vi "HFRR ADV v041.vi"() -> ()   [LabVIEW 2025] (continued)
            n2218 = Delete From Array(array=w2421, index=0) -> (array with subset deleted=w2408:dbl[])  [unwired: 1 in, 1 out]
            n2219 = Delete From Array(array=w2461, index=0) -> (array with subset deleted=w2432:dbl[])  [unwired: 1 in, 1 out]
            n2220 = Delete From Array(array=w2539, index=0) -> (array with subset deleted=w2494:dbl[])  [unwired: 1 in, 1 out]
            n2221 = Delete From Array(array=w2505, index=0) -> (array with subset deleted=w2490:dbl[])  [unwired: 1 in, 1 out]
            "array w/ subset deleted" <- w2490
            n2222 = Delete From Array(array=w2536, index=0) -> (array with subset deleted=w2537:dbl[])  [unwired: 1 in, 1 out]
            n2223 = call-poly <vilib>:"Mean.vi"("X"=w2432) -> ("mean"=→"КОФ2 2":dbl)  [unwired: 1 out]
            n2224 = call-poly <vilib>:"Mean.vi"("X"=w2494) -> ("mean"=→"КОФ1":dbl)  [unwired: 1 out]
            n2225 = Bundle "Bundle"(w2409, w2408) -> (w2414:cluster{dbl[], dbl[]})  [unwired: 1 in]
            n2226 = Bundle "Bundle"(w2409, w2537) -> (w2401:cluster{dbl[], dbl[]})  [unwired: 1 in]
            n2227 = Delete From Array(array=w2416, index=0) -> (array with subset deleted=w2404:dbl[])  [unwired: 1 in, 1 out]
            n2228 = Delete From Array(array=w2417, index=0) -> (array with subset deleted=w2406:dbl[])  [unwired: 1 in, 1 out]
            n2229 = Delete From Array(array=w2527, index=0) -> (array with subset deleted=w2528:dbl[])  [unwired: 1 in, 1 out]
            n2230 = Delete From Array(array=w2415, index=0) -> (array with subset deleted=w2402:dbl[])  [unwired: 1 in, 1 out]
            n2231 = Delete From Array(array=w2509, index=0) -> (array with subset deleted=w2510:dbl[])  [unwired: 1 in, 1 out]
            n2232 = Delete From Array(array=w2534, index=0) -> (array with subset deleted=w2440:dbl[])  [unwired: 1 in, 1 out]
            n2233 = Delete From Array(array=w2480, index=0) -> (array with subset deleted=w2436:dbl[])  [unwired: 1 in, 1 out]
            n2234 = Delete From Array(array=w2516, index=0) -> (array with subset deleted=w2438:dbl[])  [unwired: 1 in, 1 out]
            n2235 = Delete From Array(array=w2476, index=0) -> (array with subset deleted=w2434:dbl[])  [unwired: 1 in, 1 out]
            n2236 = Delete From Array(array=w2525, index=0) -> (array with subset deleted=w2439:dbl[])  [unwired: 1 in, 1 out]
            n2237 = Delete From Array(array=w2478, index=0) -> (array with subset deleted=w2435:dbl[])  [unwired: 1 in, 1 out]
            n2238 = Delete From Array(array=w2459, index=0) -> (array with subset deleted=w2431:dbl[])  [unwired: 1 in, 1 out]
            n2239 = Delete From Array(array=w2503, index=0) -> (array with subset deleted=w2489:dbl[])  [unwired: 1 in, 1 out]
            n2240 = Delete From Array(array=w2530, index=0) -> (array with subset deleted=w2491:dbl[])  [unwired: 1 in, 1 out]
            n2241 = Delete From Array(array=w2507, index=0) -> (array with subset deleted=w2437:dbl[])  [unwired: 1 in, 1 out]
            n2242 = Delete From Array(array=w2474, index=0) -> (array with subset deleted=w2433:dbl[])  [unwired: 1 in, 1 out]
            n2243 = Delete From Array(array=w2455, index=0) -> (array with subset deleted=w2429:dbl[])  [unwired: 1 in, 1 out]
            n2244 = Delete From Array(array=w2499, index=0) -> (array with subset deleted=w2487:dbl[])  [unwired: 1 in, 1 out]
            n2245 = Delete From Array(array=w2512, index=0) -> (array with subset deleted=w2492:dbl[])  [unwired: 1 in, 1 out]
            n2246 = Delete From Array(array=w2522, index=0) -> (array with subset deleted=w2405:dbl[])  [unwired: 1 in, 1 out]
            n2247 = Delete From Array(array=w2532, index=0) -> (array with subset deleted=w2407:dbl[])  [unwired: 1 in, 1 out]
            n2248 = Delete From Array(array=w2514, index=0) -> (array with subset deleted=w2403:dbl[])  [unwired: 1 in, 1 out]
            n2249 = Bundle "Bundle"(w2409, w2440) -> (w2427:cluster{dbl[], dbl[]})  [unwired: 1 in]
            n2250 = Bundle "Bundle"(w2409, w2494) -> (w2428:cluster{dbl[], dbl[]})  [unwired: 1 in]
            n2251 = Bundle "Bundle"(w2440, w2436) -> (w2442:cluster{dbl[], dbl[]})  [unwired: 1 in]
            n2252 = Bundle "Bundle"(w2405, w2404) -> (w2412:cluster{dbl[], dbl[]})  [unwired: 1 in]
            n2253 = Bundle "Bundle"(w2438, w2434) -> (w2444:cluster{dbl[], dbl[]})  [unwired: 1 in]
            n2254 = Bundle "Bundle"(w2405, w2438) -> (w2548:cluster{dbl[], dbl[]})  [unwired: 1 in]
            n2255 = Bundle "Bundle"(w2405, w2434) -> (w2472:cluster{dbl[], dbl[]})  [unwired: 1 in]
            n2256 = Bundle "Bundle"(w2405, w2493) -> (w2558:cluster{dbl[], dbl[]})  [unwired: 1 in]
            n2257 = Bundle "Bundle"(w2405, w2488) -> (w2496:cluster{dbl[], dbl[]})  [unwired: 1 in]
            n2258 = Bundle "Bundle"(w2405, w2519) -> (w2543:cluster{dbl[], dbl[]})  [unwired: 1 in]
            n2259 = Bundle "Bundle"(w2439, w2435) -> (w2443:cluster{dbl[], dbl[]})  [unwired: 1 in]
            n2260 = Bundle "Bundle"(w2407, w2406) -> (w2413:cluster{dbl[], dbl[]})  [unwired: 1 in]
            n2261 = Bundle "Bundle"(w2407, w2439) -> (w2550:cluster{dbl[], dbl[]})  [unwired: 1 in]
            n2262 = Bundle "Bundle"(w2407, w2435) -> (w2473:cluster{dbl[], dbl[]})  [unwired: 1 in]
            n2263 = Bundle "Bundle"(w2407, w2489) -> (w2497:cluster{dbl[], dbl[]})  [unwired: 1 in]
            n2264 = Bundle "Bundle"(w2407, w2491) -> (w2559:cluster{dbl[], dbl[]})  [unwired: 1 in]
            n2265 = Bundle "Bundle"(w2407, w2528) -> (w2541:cluster{dbl[], dbl[]})  [unwired: 1 in]
            n2266 = Bundle "Bundle"(w2437, w2433) -> (w2445:cluster{dbl[], dbl[]})  [unwired: 1 in]
            n2267 = Bundle "Bundle"(w2403, w2402) -> (w2411:cluster{dbl[], dbl[]})  [unwired: 1 in]
            n2268 = Bundle "Bundle"(w2403, w2437) -> (w2549:cluster{dbl[], dbl[]})  [unwired: 1 in]
            n2269 = Bundle "Bundle"(w2403, w2433) -> (w2471:cluster{dbl[], dbl[]})  [unwired: 1 in]
            n2270 = Bundle "Bundle"(w2403, w2487) -> (w2495:cluster{dbl[], dbl[]})  [unwired: 1 in]
            n2271 = Bundle "Bundle"(w2403, w2492) -> (w2557:cluster{dbl[], dbl[]})  [unwired: 1 in]
            n2272 = Bundle "Bundle"(w2403, w2510) -> (w2542:cluster{dbl[], dbl[]})  [unwired: 1 in]
            n2273 = call-poly <vilib>:"Mean.vi"("X"=w2490) -> ("mean"=→"CP1":dbl)  [unwired: 1 out]
            n2274 = call-poly <vilib>:"Mean.vi"("X"=w2431) -> ("mean"=→"КОФ2 3":dbl)  [unwired: 1 out]
            n2275 = call-poly <vilib>:"Mean.vi"("X"=w2489) -> ("mean"=→"CP2":dbl)  [unwired: 1 out]
            n2276 = call-poly <vilib>:"Mean.vi"("X"=w2491) -> ("mean"=→"КОФ2":dbl)  [unwired: 1 out]
            n2277 = call-poly <vilib>:"Mean.vi"("X"=w2429) -> ("mean"=→"КОФ2 5":dbl)  [unwired: 1 out]
            n2278 = call-poly <vilib>:"Mean.vi"("X"=w2487) -> ("mean"=→"CP4":dbl)  [unwired: 1 out]
            n2279 = call-poly <vilib>:"Mean.vi"("X"=w2492) -> ("mean"=→"КОФ4":dbl)  [unwired: 1 out]
            n2280 = Bundle "Bundle"(w2409, w2436) -> (w2400:cluster{dbl[], dbl[]})  [unwired: 1 in]
            n2281 = Bundle "Bundle"(w2409, w2490) -> (w2423:cluster{dbl[], dbl[]})  [unwired: 1 in]
            n2282 = Build Array "Build Array"(w2400, w2423) -> (w2426:cluster{dbl[], dbl[]}[])
            "XY Graph 17" <- w2426
            n2283 = Build Array "Build Array"(w2414, w2413, w2412, w2411) -> (→"Frequency ( Hz )":cluster{dbl[], dbl[]}[])
            n2284 = Build Array "Build Array"(w2442, w2443, w2444, w2445) -> (→"Air Temp ( °C ) vs Humidity ( % RH )":cluster{dbl[], dbl[]}[])
            n2285 = Build Array "Build Array"(w2427, w2550, w2548, w2549) -> (→"Air Temperature  ( °C )":cluster{dbl[], dbl[]}[])
            n2286 = Build Array "Build Array"(w2400, w2473, w2472, w2471) -> (→"Humidity ( %RH )":cluster{dbl[], dbl[]}[])
            n2287 = Build Array "Build Array"(w2428, w2559, w2558, w2557) -> (→"Coefficient Of Friction":cluster{dbl[], dbl[]}[])
            n2288 = Build Array "Build Array"(w2423, w2497, w2496, w2495) -> (→"Sample Temperature ( °C )":cluster{dbl[], dbl[]}[])
            n2289 = Build Array "Build Array"(w2401, w2541, w2543, w2542) -> (→"XY Graph 13":cluster{dbl[], dbl[]}[])
            n2290 = Bundle "Bundle"(w2409, w2432) -> (w2454:cluster{dbl[], dbl[]})  [unwired: 1 in]
            n2291 = Bundle "Bundle"(w2405, w2430) -> (w2452:cluster{dbl[], dbl[]})  [unwired: 1 in]
            n2292 = Bundle "Bundle"(w2407, w2431) -> (w2453:cluster{dbl[], dbl[]})  [unwired: 1 in]
            n2293 = Bundle "Bundle"(w2403, w2429) -> (w2451:cluster{dbl[], dbl[]})  [unwired: 1 in]
            n2294 = Build Array "Build Array"(w2454, w2453, w2452, w2451) -> (→"Stroke ( mm )":cluster{dbl[], dbl[]}[])
            n2295 = local write "XY Graph 16"(w2426) -> ()
          }
          frame #2 {
          }
          frame #3 {
            n2296 = local write "Numeric 8"(0 ("Numeric 8")) -> ()
            n2297 = local write "Numeric 11"(0 ("Numeric 11")) -> ()
            n2298 = local write "Numeric 12"(0 ("Numeric 12")) -> ()
            n2299 = local write "Numeric 13"(0 ("Numeric 13")) -> ()
            n2300 = property on="OPEN" class="Bool (strict)"("Visible"=TRUE) -> ()  [unwired: 2 in, 2 out]
            n2301 = local read "String Control 2"() -> (w2726:string)
            n2302 = local read "String Control 4"() -> (w2725:string)
            n2303 = local read "String Control 6"() -> (w2724:string)
            n2304 = local read "String Control 8"() -> (w2723:string)
            n2305 = Match Pattern(string=w2726, regular expression="Samples / cycle :- ") -> (after substring=w2740:string)  [unwired: 1 in, 3 out]
            n2306 = Match Pattern(string=w2726, regular expression="Frequency :- ") -> (after substring=w2759:string)  [unwired: 1 in, 3 out]
            n2307 = Match Pattern(string=w2725, regular expression="Samples / cycle :- ") -> (after substring=w2736:string)  [unwired: 1 in, 3 out]
            n2308 = Match Pattern(string=w2725, regular expression="Frequency :- ") -> (after substring=w2754:string)  [unwired: 1 in, 3 out]
            n2309 = Match Pattern(string=w2724, regular expression="Samples / cycle :- ") -> (after substring=w2732:string)  [unwired: 1 in, 3 out]
            n2310 = Match Pattern(string=w2724, regular expression="Frequency :- ") -> (after substring=w2749:string)  [unwired: 1 in, 3 out]
            n2311 = Match Pattern(string=w2723, regular expression="Samples / cycle :- ") -> (after substring=w2728:string)  [unwired: 1 in, 3 out]
            n2312 = Match Pattern(string=w2723, regular expression="Frequency :- ") -> (after substring=w2744:string)  [unwired: 1 in, 3 out]
            n2313 = String Subset(string=w2740, length (rest)=6 ("length (rest)")) -> (substring=w2742:string)  [unwired: 1 in]
            n2314 = String Subset(string=w2759, length (rest)=9 ("length (rest)")) -> (substring=w2761:string)  [unwired: 1 in]
            n2315 = String Subset(string=w2736, length (rest)=6 ("length (rest)")) -> (substring=w2738:string)  [unwired: 1 in]
            n2316 = String Subset(string=w2754, length (rest)=9 ("length (rest)")) -> (substring=w2756:string)  [unwired: 1 in]
            n2317 = String Subset(string=w2732, length (rest)=6 ("length (rest)")) -> (substring=w2734:string)  [unwired: 1 in]
            n2318 = String Subset(string=w2749, length (rest)=9 ("length (rest)")) -> (substring=w2751:string)  [unwired: 1 in]
            n2319 = String Subset(string=w2728, length (rest)=6 ("length (rest)")) -> (substring=w2730:string)  [unwired: 1 in]
            n2320 = String Subset(string=w2744, length (rest)=9 ("length (rest)")) -> (substring=w2746:string)  [unwired: 1 in]
            n2321 = Fract/Exp String To Number(string=w2742) -> (number=w2722:dbl)  [unwired: 3 in, 1 out]
            n2322 = Fract/Exp String To Number(string=w2761) -> (number=w2762:dbl)  [unwired: 3 in, 1 out]
            n2323 = Fract/Exp String To Number(string=w2738) -> (number=w2721:dbl)  [unwired: 3 in, 1 out]
            n2324 = Fract/Exp String To Number(string=w2756) -> (number=w2757:dbl)  [unwired: 3 in, 1 out]
            n2325 = Fract/Exp String To Number(string=w2734) -> (number=w2720:dbl)  [unwired: 3 in, 1 out]
            n2326 = Fract/Exp String To Number(string=w2751) -> (number=w2752:dbl)  [unwired: 3 in, 1 out]
            n2327 = Fract/Exp String To Number(string=w2730) -> (number=w2719:dbl)  [unwired: 3 in, 1 out]
            n2328 = Fract/Exp String To Number(string=w2746) -> (number=w2747:dbl)  [unwired: 3 in, 1 out]
            n2329 = local write "sample1"(w2722) -> ()
            n2330 = local write "freq1"(w2762) -> ()
            n2331 = local write "sample2"(w2721) -> ()
            n2332 = local write "freq2"(w2757) -> ()
            n2333 = local write "sample3"(w2720) -> ()
            n2334 = local write "freq3"(w2752) -> ()
            n2335 = local write "sample4"(w2719) -> ()
            n2336 = local write "freq 4"(w2747) -> ()
          }
        }
      }
    }
    n2337 = case shown="True" w2320 {
      selector: w2320 -> [_ w2339]
      frame False {
      }
      frame True {
        n2338 = Not(x=w2339) -> (.not. x?=w2335:bool)
        n2339 = local write "service 3"(w2335) -> ()
        n2340 = local write "OPEN 6"(w2335) -> ()
        n2341 = call <vilib>:"System Exec.vi"("wait until completion? (T)"=TRUE, "command line"="C:\\LAB-IQ\\Scar View.exe") -> ("error out"=→"error out 5":errorcluster)  [unwired: 6 in, 3 out]
      }
    }
    n2342 = case shown="\"Acquire\", Default" w2329 {
      frame "Acquire", Default {
        # "Elapsed time\ncof\nstroke\nAir temp\nTemp\nHumidity"
        n2343 = disable-structure shown="Disabled" {
          frame Disabled {
            n2344 = local read "Flag"() -> (w3038:dbl)
            n2345 = local read "RUN"() -> (w3035:bool)
            n2346 = Not(x=w3035) -> (.not. x?=w3034:bool)
            n2347 = Equal?(x=w3038, y=10.0) -> (x = y?=w3036:bool)
            n2348 = And(x=w3036, y=w3034) -> (x .and. y?=w3033:bool)
            n2349 = case shown="True" w3033 {
              frame False {
              }
              frame True {
                w3039 = FALSE ("Heater Button")
                n2350 = local write "Humidity"(w3039) -> ()
                n2351 = local write "Heater Button"(w3039) -> ()
              }
            }
          }
          frame Enabled {
          }
        }
        n2352 = disable-structure shown="Disabled" {
          frame Disabled {
            n2353 = case shown="True" {
              selector: _ -> [_ _]
              frame False {
              }
              frame True {
                w3084 = TRUE ("Heater")
                n2354 = local write "Humidity"(w3084) -> ()
                n2355 = local write "Heater Button"(w3084) -> ()
                n2356 = local read "TEST STANDARD"() -> (w3087:T3)
                n2357 = local read "TEST STANDARD"() -> (w3082:T3)
                n2358 = Equal?(x=w3087, y=enum16{"ASTM D6079", "ISO 12156", "Custom"}."ISO 12156" ("Test Standard")) -> (x = y?=w3085:bool)
                n2359 = Equal?(x=w3082, y=enum16{"ASTM D6079", "ISO 12156", "Custom"}."ASTM D6079" ("Test Standard")) -> (x = y?=w3081:bool)
                n2360 = case shown="True" w3085 {
                  frame False {
                  }
                  frame True {
                    n2361 = local write "airtempflg"(FALSE ("airtempflg")) -> ()
                    n2362 = local write item#-1(TRUE ("Heater")) -> ()
                  }
                }
                n2363 = case shown="True" w3081 {
                  frame False {
                  }
                  frame True {
                    n2364 = local write "airtempflg"(TRUE ("airtempflg")) -> ()
                    n2365 = local write item#-1(FALSE ("Heater")) -> ()
                  }
                }
              }
            }
          }
          frame Enabled {
          }
        }
        n2366 = stacked-sequence {
          frame #0 {
            n2367 = case shown="True" "RST FF" {
              frame False {
              }
              frame True {
                w3101 = 0.0 ("X Scale.Range:Maximum")
                n2368 = property on="Frictional Force ( N )" class="WFChart (strict)"("XScale.Maximum"=600.0 ("X Scale.Range:Maximum"), "XScale.Minimum"=w3101, "YScale.Maximum"=10.0 ("Y Scale.Range:Maximum"), "YScale.Minimum"=w3101) -> ()  [unwired: 2 in, 2 out]
              }
            }
          }
          frame #1 {
            n2369 = case shown="True" "RST TEMP" {
              frame False {
              }
              frame True {
                n2370 = property on="Temperature ( Deg C )" class="WFChart (strict)"("XScale.Minimum"=0.0 ("X Scale.Range:Minimum"), "XScale.Maximum"=600.0 ("X Scale.Range:Maximum"), "YScale.Minimum"=0.0 ("Y Scale.Range:Minimum"), "YScale.Maximum"=100.0 ("Y Scale.Range:Maximum")) -> ()  [unwired: 2 in, 2 out]
              }
            }
          }
          frame #2 {
            n2371 = case shown="True" "RSTCOF" {
              frame False {
              }
              frame True {
                n2372 = property on="Coefficient of Friction" class="WFChart (strict)"("XScale.Minimum"=0.0 ("X Scale.Range:Minimum"), "XScale.Maximum"=600.0 ("X Scale.Range:Maximum"), "YScale.Maximum"=1.0 ("X Scale.Range:Minimum"), "YScale.Minimum"=0.0 ("X Scale.Range:Minimum")) -> ()  [unwired: 2 in, 2 out]
              }
            }
          }
          frame #3 {
            n2373 = case shown="True" "RSTCOF 2" {
              frame False {
              }
              frame True {
                (unwired) 100.0 ("Y Scale.Range:Maximum")
                (unwired) 0.0 ("Y Scale.Range:Minimum")
                (unwired) 600.0 ("X Scale.Range:Maximum")
                (unwired) 0.0 ("X Scale.Range:Minimum")
              }
            }
          }
          frame #4 {
            n2374 = case shown="True" "RSTCOF 3" {
              frame False {
              }
              frame True {
                n2375 = property on="Electrical Contact Resistance ( % )" class="WFChart (strict)"("XScale.Minimum"=0.0 ("X Scale.Range:Minimum"), "XScale.Maximum"=600.0 ("X Scale.Range:Maximum"), "YScale.Minimum"=0.0 ("Y Scale.Range:Minimum"), "YScale.Maximum"=100.0 ("Y Scale.Range:Maximum")) -> ()  [unwired: 2 in, 2 out]
              }
            }
          }
        }
        n2376 = local read "RUN"() -> (w3028:bool)
        n2377 = case shown="False" w3028 {
          frame False {
          }
          frame True {
          }
        }
        n2378 = local read "RUN"() -> (w3032:bool)
        n2379 = case shown="False" w3032 {
          tunnel: [FALSE ("TEST RUNNING") TRUE ("TEST RUNNING")] -> w3031
          frame False {
            w3120 = 0.0 ("Flag")
            n2380 = local write "Elapsed time"(0.0 ("elapsedtime")) -> ()
            n2381 = local write "Time Remaining"(w3120) -> ()
            n2382 = local write "Flag"(w3120) -> ()
            n2383 = local write "Remaining Time"(w3120) -> ()
          }
          frame True {
            n2384 = local write "Flag"(10.0 ("Flag")) -> ()
          }
        }
        n2385 = local read "AIR TEMP"() -> (w3026:dbl)
        n2386 = Greater Or Equal?(x=w3026, y=15.0) -> (x >= y?=w3027:bool)
        "powstat" <- w3027
        n2387 = case shown="True" "Save & Continue" {
          frame False {
          }
          frame True {
            n2388 = local read "USER ID"() -> (w3424:string)
            n2389 = local read "FILE"() -> (w3432:string)
            n2390 = String Length(string=w3432) -> (length=w3430:i32)
            n2391 = String Length(string=w3424) -> (length=w3427:i32)
            n2392 = Greater?(x=w3430, y=0) -> (0:w3429:bool)
            n2393 = Greater?(x=w3427, y=0) -> (0:w3426:bool)
            n2394 = And(x=w3429, y=w3426) -> (x .and. y?=w3425:bool)
            n2395 = case shown="True" w3425 {
              frame False {
                n2396 = stacked-sequence {
                  frame #0 {
                    n2397 = One Button Dialog(message="Please Enter a File Name and Operator ID to save data !", button name ("OK")="Ok") -> ()  [unwired: 1 out]
                  }
                  frame #1 {
                    n2398 = local write "Save & Continue"(FALSE ("OK Button")) -> ()
                  }
                }
                n2399 = local write "Save & Continue"(FALSE ("OK Button")) -> ()
              }
              frame True {
                n2400 = stacked-sequence {
                  frame #0 {
                    n2401 = local read "FILE"() -> (w3438:string)
                    n2402 = call "file check.vi"("file name in"=w3438) -> ("file name out"=w3437:string)  [unwired: 9 in, 1 out]
                    n2403 = call <vilib>:"Application Directory.vi"() -> ("Application Directory"=w3448:path)
                    n2404 = Build Path(base path=w3448, name or relative path="data") -> (appended path=w3447:path)
                    n2405 = call <vilib>:"Trim Whitespace.vi"("string"=w3437) -> ("trimmed string"=w3445:string)  [unwired: 1 in]
                    n2406 = call <vilib>:"Trim Whitespace.vi"("string"=w3437) -> ("trimmed string"=w3446:string)  [unwired: 1 in]
                    n2407 = List Folder(path=w3447) -> (folder names=w3443:string[])  [unwired: 3 in, 3 out]
                    n2408 = Match Pattern(string=w3445, regular expression="_(") -> (before substring=w3442:string)  [unwired: 1 in, 3 out]
                    n2409 = for {
                      tunnel: w3443 -> [w3457] mode=indexing
                      tunnel: w3442 -> [w3455]
                      shift-right: [w3453] -> w3440
                      shift-left: bool[] [] -> [w3454]
                      n2410 = Match Pattern(string=w3457, regular expression="_(") -> (before substring=w3456:string)  [unwired: 1 in, 3 out]
                      n2411 = Equal?(x=w3456, y=w3455) -> (x = y?=w3452:bool)
                      n2412 = case shown="True" w3452 {
                        tunnel: w3452 -> [_ w3460]
                        tunnel: w3454 -> [w3459 w3462]
                        tunnel: [w3459 w3461] -> w3453
                        frame False {
                        }
                        frame True {
                          n2413 = Insert Into Array(array=w3462, new element=w3460) -> (w3461:bool[])  [unwired: 1 in]
                        }
                      }
                    }
                    n2414 = Equal?(x=w3443, y=w3442) -> (x = y?=w3451:bool[])
                    n2415 = Or Array Elements(Boolean array=w3451) -> (logical OR=w3450:bool)
                    n2416 = Array Size(array=w3440) -> (size(s)=w3439:i32)
                    n2417 = case shown="True" w3450 {
                      tunnel: w3446 -> [_ w3470]
                      tunnel: w3439 -> [_ w3463]
                      frame False {
                      }
                      frame True {
                        n2418 = Number To Decimal String(number=w3463) -> (decimal integer string=w3466:string)  [unwired: 1 in]
                        n2419 = Search/Split String(string=w3470, search string/char (-)="_(" ("regular expression")) -> (substring before match=w3468:string)  [unwired: 1 in, 2 out]
                        n2420 = Concatenate Strings(w3468, "_(" ("regular expression"), w3466, ")" ("regular expression")) -> (w3464:string)
                        n2421 = local write "FILE"(w3464) -> ()
                      }
                    }
                  }
                  frame #1 {
                    w3473 = 0.0
                    w3486 = cluster{"y":dbl, dbl, "y":dbl}[] [] ("History Data")
                    w3487 = FALSE ("Heater Button")
                    (unwired) ")!" ("string")
                    (unwired) ")" ("string")
                    w3485 = dbl[] [] ("History Data")
                    w3491 = "\r"
                    # "C:\\WinDucom\\Data\\"
                    # "C:\\LAB-IQ-NXT\\data"
                    n2422 = local write "Humidity ( %RH )"(w3473) -> ()
                    n2423 = local write "Frequency ( Hz )"(w3473) -> ()
                    n2424 = local write "Stroke 3"(w3473) -> ()
                    n2425 = local write "speedop"(0.0 ("PIDclk 2")) -> ()
                    n2426 = local write "Set Temp 2"(65.0 ("Set Temp 2")) -> ()
                    n2427 = local write "AIR TEMP"(w3473) -> ()
                    n2428 = local write "clk"(0.0 ("clk")) -> ()
                    n2429 = local write "Stroke 4"(w3473) -> ()
                    n2430 = local write "COF 2"(w3473) -> ()
                    n2431 = local write "TEMP"(w3473) -> ()
                    n2432 = local write "ecr 3"(w3473) -> ()
                    n2433 = local write "FF 3"(w3473) -> ()
                    n2434 = local write "FF 2"(w3473) -> ()
                    n2435 = property on="Coefficient of Friction" class="WFChart (strict)"("History Data"=w3485) -> ()  [unwired: 2 in, 2 out]
                    n2436 = property on="Coefficient of Friction" class="WFChart (strict)"("History Data"=w3485) -> ()  [unwired: 2 in, 2 out]
                    n2437 = property on="Frictional Force ( N )" class="WFChart (strict)"("History Data"=w3485) -> ()  [unwired: 2 in, 2 out]
                    n2438 = property on="Electrical Contact Resistance ( % )" class="WFChart (strict)"("History Data"=w3485) -> ()  [unwired: 2 in, 2 out]
                    n2439 = property on="Electrical Contact Resistance ( % )" class="WFChart (strict)"("History Data"=w3485) -> ()  [unwired: 2 in, 2 out]
                    n2440 = property on="Temperature ( Deg C )" class="WFChart (strict)"("History Data"=w3485) -> ()  [unwired: 2 in, 2 out]
                    n2441 = property on="Frictional Force ( N )" class="WFChart (strict)"("History Data"=w3485) -> ()  [unwired: 2 in, 2 out]
                    n2442 = property on="Coefficient of Friction" class="WFChart (strict)"("History Data"=w3485) -> ()  [unwired: 2 in, 2 out]
                    n2443 = property on="Frictional Force ( N )" class="WFChart (strict)"("History Data"=w3485) -> ()  [unwired: 2 in, 2 out]
                    n2444 = property on="Electrical Contact Resistance ( % )" class="WFChart (strict)"("History Data"=w3485) -> ()  [unwired: 2 in, 2 out]
                    n2445 = property on="Temperature ( Deg C )" class="WFChart (strict)"("History Data"=w3485) -> ()  [unwired: 2 in, 2 out]
                    n2446 = property on="Stroke ( mm )" class="WFChart (strict)"("History Data"=w3486) -> ()  [unwired: 2 in, 2 out]
                    n2447 = property on="Stroke ( mm )" class="WFChart (strict)"("History Data"=w3486) -> ()  [unwired: 2 in, 2 out]
                    n2448 = local write "Humidity"(w3487) -> ()
                    n2449 = local write "Heater Button"(w3487) -> ()
                    n2450 = local read "FILE"() -> (w3481:string)
                    n2451 = disable-structure shown="Enabled" {
                      disable-tunnel: [w3525 _] -> w3472
                      frame Enabled {
                        n2452 = local read "NORMAL LOAD"() -> (w3525:dbl)
                      }
                      frame Disabled {
                      }
                    }
                    n2453 = call "file check.vi"("file name in"=w3481) -> ("error out"=w3484:errorcluster, "file name out"=w3478:string)  [unwired: 9 in]
                    n2454 = call "FILE PATH CREATION.vi"("error in"=w3484, "FILE NAME :"=w3478) -> ("FILE OUT"=w3477:path)  [unwired: 8 in, 1 out]
                    n2455 = Concatenate Strings(w3478, ".dgf" ("Substring")) -> (w3483:string)
                    n2456 = Concatenate Strings(w3478, ".duf" ("Substring")) -> (w3479:string)
                    n2457 = Multiply(x=w3472, y=1.0) -> (x*y=w3504:dbl)
                    n2458 = Build Path(base path=w3477, name or relative path=w3483) -> (appended path=w3476:path)
                    n2459 = Build Path(base path=w3477, name or relative path=w3479) -> (appended path=w3475:path)
                    n2460 = Number To Fractional String(number=w3504, width (-)=i16 5, precision (6)=i16 2) -> (F-format string=w3512:string)  [unwired: 1 in]
                    n2461 = local read "tested by"() -> (w3471:string)
                    n2462 = local read "Fuel Discription :"() -> (w3500:string)
                    n2463 = local read "Batch Ref Num :"() -> (w3489:string)
                    n2464 = Get Date/Time String(date format (0)=enum16{"short", "long", "abbreviated"}."short") -> (date string=w3523:string, time string=w3520:string)  [unwired: 2 in]
                    n2465 = local read "Remarks :"() -> (w3499:string)
                    n2466 = Concatenate Strings("Load :- " ("Substring"), w3512, " grams ," ("Substring")) -> (w3511:string)
                    n2467 = local read "String 41"() -> (w3492:string)
                    n2468 = Concatenate Strings(w3500) -> (w3501:string)
                    n2469 = Concatenate Strings(w3489) -> (w3488:string)
                    n2470 = Concatenate Strings(w3471) -> (w3495:string)
                    n2471 = Concatenate Strings("(" ("Substring"), w3523, ")" ("Substring"), w3520) -> (w3494:string)
                    "concatenated string" <- w3494
                    n2472 = Concatenate Strings(w3499, "," ("string")) -> (w3498:string)
                    n2473 = Concatenate Strings("  TIME;      COF;       STROKE;     AIR TEMP;  TEMP;  HUMIDITY;  ECR; PID-OUT; FREQUENCY" ("Substring"), "\r") -> (w3507:string)
                    n2474 = Concatenate Strings(w3492, w3491, "Fuel Discription :-" ("Substring"), w3501, w3491, w3511, w3491, "Batch Ref Num :-" ("Substring"), w3488, w3491, " Remarks :- " ("Substring"), w3498, w3491, " Date :- " ("Substring"), w3494, w3491, "Tested By :-" ("Substring"), w3495) -> (w3505:string)
                    "REMARKS" <- w3505
                    n2475 = call <vilib>:"Write Characters To File.vi"("append to file? (new file:F)"=FALSE, "character string"=w3507, "file path (dialog if empty)"=w3476) -> ()  [unwired: 2 in, 1 out]
                    n2476 = call <vilib>:"Write Characters To File.vi"("append to file? (new file:F)"=FALSE, "character string"=w3505, "file path (dialog if empty)"=w3475) -> ()  [unwired: 2 in, 1 out]
                  }
                  frame #2 {
                    n2477 = local write "Cycles elapsed"(0 ("Cycles elapsed")) -> ()
                    n2478 = local write "cyclecount"(0 ("cyclecount")) -> ()
                    n2479 = local write "Save & Continue"(FALSE ("OK")) -> ()
                    n2480 = local write "autostrtflg"(TRUE ("autostrtflg")) -> ()
                    n2481 = local write "Save"(FALSE ("Save")) -> ()
                    n2482 = Get Date/Time In Seconds() -> (seconds since 1Jan1904=w3530:timestamp)
                    n2483 = To Double Precision Float(number=w3530) -> (double precision float=w3529:dbl)
                    n2484 = local write "acq timer"(w3529) -> ()
                    n2485 = One Button Dialog(message="Please ensure sample is mounted properly and machine is ready in all aspects for testing !", button name ("OK")="Ok") -> ()  [unwired: 1 out]
                  }
                  frame #3 {
                    n2486 = stacked-sequence {
                      frame #0 {
                        n2487 = local write "Main Dashboard Buttons"(T1."Dashboard" ("Main Dashboard Buttons")) -> ()
                        n2488 = local write "Main Tab"(T2."Acquire" ("Main Tab")) -> ()
                      }
                      frame #1 {
                        n2489 = local write "EVENT LOG"("" ("EVENT LOG")) -> ()
                      }
                      frame #2 {
                        n2490 = Wait (ms)(milliseconds to wait=u32 50) -> ()  [unwired: 1 out]
                      }
                      frame #3 {
                        n2491 = disable-structure shown="Disabled" {
                          frame Disabled {
                            n2492 = local read "EVENT LOG"() -> (w3542:string)
                            n2493 = call "Event Log.vi"("Content"="Test Details", "EVENT LOG"=w3542) -> ("EVENT LOG"=w3541:string)  [unwired: 8 in, 1 out]
                            n2494 = local write "EVENT LOG"(w3541) -> ()
                          }
                          frame Enabled {
                          }
                        }
                      }
                      frame #4 {
                        n2495 = Wait (ms)(milliseconds to wait=u32 50) -> ()  [unwired: 1 out]
                      }
                      frame #5 {
                        n2496 = local read "FILE"() -> (w3544:string)
                        n2497 = Concatenate Strings("File Name :" ("Content"), w3544) -> (w3545:string)
                        n2498 = local read "EVENT LOG"() -> (w3548:string)
                        n2499 = call "Event Log.vi"("Content"=w3545, "EVENT LOG"=w3548) -> ("EVENT LOG"=w3547:string)  [unwired: 8 in, 1 out]
                        n2500 = local write "EVENT LOG"(w3547) -> ()
                      }
                      frame #6 {
                        n2501 = Wait (ms)(milliseconds to wait=u32 50) -> ()  [unwired: 1 out]
                      }
                      frame #7 {
                        n2502 = local read "Batch Ref Num :"() -> (w3550:string)
                        n2503 = Concatenate Strings("Batch Ref No :" ("Content"), w3550) -> (w3551:string)
                        n2504 = local read "EVENT LOG"() -> (w3554:string)
                        n2505 = call "Event Log.vi"("Content"=w3551, "EVENT LOG"=w3554) -> ("EVENT LOG"=w3553:string)  [unwired: 8 in, 1 out]
                        n2506 = local write "EVENT LOG"(w3553) -> ()
                      }
                      frame #8 {
                        n2507 = Wait (ms)(milliseconds to wait=u32 50) -> ()  [unwired: 1 out]
                      }
                      frame #9 {
                        n2508 = local read "tested by"() -> (w3556:string)
                        n2509 = Concatenate Strings("Tested By :" ("Content"), w3556) -> (w3557:string)
                        n2510 = local read "EVENT LOG"() -> (w3560:string)
                        n2511 = call "Event Log.vi"("Content"=w3557, "EVENT LOG"=w3560) -> ("EVENT LOG"=w3559:string)  [unwired: 8 in, 1 out]
                        n2512 = local write "EVENT LOG"(w3559) -> ()
                      }
                      frame #10 {
                        n2513 = Wait (ms)(milliseconds to wait=u32 50) -> ()  [unwired: 1 out]
                      }
                      frame #11 {
                        n2514 = local read "TEST STANDARD"() -> (w3563:T3)
                        n2515 = case shown="\"ASTM D6079\", Default" w3563 {
                          tunnel: ["ASTM D6079" "ISO 12156" "CEC F-096-A-06" "Custom"] -> w3562
                          frame "ASTM D6079", Default {
                          }
                          frame "ISO 12156" {
                          }
                          frame "CEC F-096-A-06" {
                          }
                          frame "Custom" {
                          }
                        }
                        n2516 = Concatenate Strings("Test Standard :" ("Content"), w3562) -> (w3564:string)
                        n2517 = local read "EVENT LOG"() -> (w3567:string)
                        n2518 = call "Event Log.vi"("Content"=w3564, "EVENT LOG"=w3567) -> ("EVENT LOG"=w3566:string)  [unwired: 8 in, 1 out]
                        n2519 = local write "EVENT LOG"(w3566) -> ()
                      }
                      frame #12 {
                        n2520 = Wait (ms)(milliseconds to wait=u32 50) -> ()  [unwired: 1 out]
                      }
                      frame #13 {
                        n2521 = local read "Fuel Discription :"() -> (w3573:string)
                        n2522 = Concatenate Strings("Fuel Description :" ("Content"), w3573) -> (w3574:string)
                        n2523 = local read "EVENT LOG"() -> (w3577:string)
                        n2524 = call "Event Log.vi"("Content"=w3574, "EVENT LOG"=w3577) -> ("EVENT LOG"=w3576:string)  [unwired: 8 in, 1 out]
                        n2525 = local write "EVENT LOG"(w3576) -> ()
                      }
                      frame #14 {
                        n2526 = Wait (ms)(milliseconds to wait=u32 50) -> ()  [unwired: 1 out]
                      }
                      frame #15 {
                        n2527 = local read "Remarks :"() -> (w3579:string)
                        n2528 = Concatenate Strings("Remarks :" ("Content"), w3579) -> (w3580:string)
                        n2529 = local read "EVENT LOG"() -> (w3583:string)
                        n2530 = call "Event Log.vi"("Content"=w3580, "EVENT LOG"=w3583) -> ("EVENT LOG"=w3582:string)  [unwired: 8 in, 1 out]
                        n2531 = local write "EVENT LOG"(w3582) -> ()
                      }
                      frame #16 {
                        n2532 = Wait (ms)(milliseconds to wait=u32 50) -> ()  [unwired: 1 out]
                      }
                      frame #17 {
                        n2533 = local read "USER ID"() -> (w3585:string)
                        n2534 = Concatenate Strings("Operator ID :" ("Content"), w3585) -> (w3587:string)
                        n2535 = local read "EVENT LOG"() -> (w3589:string)
                        n2536 = call "Event Log.vi"("Content"=w3587, "EVENT LOG"=w3589) -> ("EVENT LOG"=w3588:string)  [unwired: 8 in, 1 out]
                        n2537 = local write "EVENT LOG"(w3588) -> ()
                      }
                      frame #18 {
                        n2538 = Wait (ms)(milliseconds to wait=u32 50) -> ()  [unwired: 1 out]
                      }
                      frame #19 {
                        n2539 = disable-structure shown="Disabled" {
                          frame Disabled {
                            n2540 = local read "EVENT LOG"() -> (w3593:string)
                            n2541 = call "Event Log.vi"("Content"="Test Parameter", "EVENT LOG"=w3593) -> ("EVENT LOG"=w3592:string)  [unwired: 8 in, 1 out]
                            n2542 = local write "EVENT LOG"(w3592) -> ()
                          }
                          frame Enabled {
                          }
                        }
                      }
                      frame #20 {
                        n2543 = Wait (ms)(milliseconds to wait=u32 50) -> ()  [unwired: 1 out]
                      }
                      frame #21 {
                        n2544 = local read "Set Hz"() -> (w3597:dbl)
                        n2545 = Number To Fractional String(number=w3597, precision (6)=i16 2) -> (F-format string=w3596:string)  [unwired: 2 in]
                        n2546 = Concatenate Strings("Set Frequency [Hz] :" ("Content"), w3596) -> (w3599:string)
                        n2547 = local read "EVENT LOG"() -> (w3601:string)
                        n2548 = call "Event Log.vi"("Content"=w3599, "EVENT LOG"=w3601) -> ("EVENT LOG"=w3600:string)  [unwired: 8 in, 1 out]
                        n2549 = local write "EVENT LOG"(w3600) -> ()
                      }
                      frame #22 {
                        n2550 = Wait (ms)(milliseconds to wait=u32 50) -> ()  [unwired: 1 out]
                      }
                      frame #23 {
                        n2551 = local read "NORMAL LOAD"() -> (w3604:dbl)
                        n2552 = Number To Fractional String(number=w3604, precision (6)=i16 2) -> (F-format string=w3605:string)  [unwired: 2 in]
                        n2553 = Concatenate Strings("Applied Load [grams] :" ("Content"), w3605) -> (w3607:string)
                        n2554 = local read "EVENT LOG"() -> (w3609:string)
                        n2555 = call "Event Log.vi"("Content"=w3607, "EVENT LOG"=w3609) -> ("EVENT LOG"=w3608:string)  [unwired: 8 in, 1 out]
                        n2556 = local write "EVENT LOG"(w3608) -> ()
                      }
                      frame #24 {
                        n2557 = Wait (ms)(milliseconds to wait=u32 50) -> ()  [unwired: 1 out]
                      }
                      frame #25 {
                        n2558 = local read "Set Strk"() -> (w3612:dbl)
                        n2559 = Number To Fractional String(number=w3612, precision (6)=i16 2) -> (F-format string=w3613:string)  [unwired: 2 in]
                        n2560 = Concatenate Strings("Set Stroke [mm] :" ("Content"), w3613) -> (w3615:string)
                        n2561 = local read "EVENT LOG"() -> (w3617:string)
                        n2562 = call "Event Log.vi"("Content"=w3615, "EVENT LOG"=w3617) -> ("EVENT LOG"=w3616:string)  [unwired: 8 in, 1 out]
                        n2563 = local write "EVENT LOG"(w3616) -> ()
                      }
                      frame #26 {
                        n2564 = Wait (ms)(milliseconds to wait=u32 50) -> ()  [unwired: 1 out]
                      }
                      frame #27 {
                        n2565 = local read "Set Temp"() -> (w3620:dbl)
                        n2566 = Number To Fractional String(number=w3620, precision (6)=i16 2) -> (F-format string=w3621:string)  [unwired: 2 in]
                        n2567 = Concatenate Strings("Set Temperature [deg C] :" ("Content"), w3621) -> (w3623:string)
                        n2568 = local read "EVENT LOG"() -> (w3625:string)
                        n2569 = call "Event Log.vi"("Content"=w3623, "EVENT LOG"=w3625) -> ("EVENT LOG"=w3624:string)  [unwired: 8 in, 1 out]
                        n2570 = local write "EVENT LOG"(w3624) -> ()
                      }
                      frame #28 {
                        n2571 = Wait (ms)(milliseconds to wait=u32 50) -> ()  [unwired: 1 out]
                      }
                      frame #29 {
                        n2572 = local read "Set Rh"() -> (w3628:dbl)
                        n2573 = Number To Fractional String(number=w3628, precision (6)=i16 2) -> (F-format string=w3629:string)  [unwired: 2 in]
                        n2574 = Concatenate Strings("Set Humidity [%RH] :" ("Content"), w3629) -> (w3631:string)
                        n2575 = local read "EVENT LOG"() -> (w3633:string)
                        n2576 = call "Event Log.vi"("Content"=w3631, "EVENT LOG"=w3633) -> ("EVENT LOG"=w3632:string)  [unwired: 8 in, 1 out]
                        n2577 = local write "EVENT LOG"(w3632) -> ()
                      }
                      frame #30 {
                        n2578 = Wait (ms)(milliseconds to wait=u32 50) -> ()  [unwired: 1 out]
                      }
                      frame #31 {
                        n2579 = local read "test time"() -> (w3636:dbl)
                        n2580 = Number To Fractional String(number=w3636, precision (6)=i16 1) -> (F-format string=w3637:string)  [unwired: 2 in]
                        n2581 = Concatenate Strings("Test Duration [mins] :" ("Content"), w3637) -> (w3639:string)
                        n2582 = local read "EVENT LOG"() -> (w3641:string)
                        n2583 = call "Event Log.vi"("Content"=w3639, "EVENT LOG"=w3641) -> ("EVENT LOG"=w3640:string)  [unwired: 8 in, 1 out]
                        n2584 = local write "EVENT LOG"(w3640) -> ()
                      }
                      frame #32 {
                        w3642 = dbl[] [] ("History Data")
                        w3643 = cluster{"y":dbl, dbl, "y":dbl}[] [] ("History Data")
                        w3644 = FALSE ("Visible")
                        n2585 = property on="Stroke ( mm )" class="WFChart (strict)"("History Data"=w3643) -> ()  [unwired: 2 in, 2 out]
                        n2586 = property on="Temperature ( Deg C )" class="WFChart (strict)"("History Data"=w3642) -> ()  [unwired: 2 in, 2 out]
                        n2587 = property on="Electrical Contact Resistance ( % )" class="WFChart (strict)"("History Data"=w3642) -> ()  [unwired: 2 in, 2 out]
                        n2588 = property on="Coefficient of Friction" class="WFChart (strict)"("History Data"=w3642) -> ()  [unwired: 2 in, 2 out]
                        n2589 = property on="Frictional Force ( N )" class="WFChart (strict)"("History Data"=w3642) -> ()  [unwired: 2 in, 2 out]
                        n2590 = property on="Coefficient of Friction" class="WFChart (strict)"("History Data"=w3642) -> ()  [unwired: 2 in, 2 out]
                        n2591 = property on="Frictional Force ( N )" class="WFChart (strict)"("History Data"=w3642) -> ()  [unwired: 2 in, 2 out]
                        n2592 = property on="Electrical Contact Resistance ( % )" class="WFChart (strict)"("History Data"=w3642) -> ()  [unwired: 2 in, 2 out]
                        n2593 = property on="Stroke ( mm )" class="WFChart (strict)"("History Data"=w3643) -> ()  [unwired: 2 in, 2 out]
                        n2594 = property on="Temperature ( Deg C )" class="WFChart (strict)"("History Data"=w3642) -> ()  [unwired: 2 in, 2 out]
                        n2595 = property on="Service Password Log" class="Str"("Visible"=w3644) -> ()  [unwired: 2 in, 2 out]
                        n2596 = property on="Password 3" class="Clust (strict)"("Visible"=w3644) -> ()  [unwired: 2 in, 2 out]
                      }
                    }
                    "TEST FILE NAM,E SAVED" <- TRUE ("TEST FILE NAM,E SAVED")
                  }
                }
              }
            }
          }
        }
        n2597 = local write "Test \nStatus"(w3031) -> ()
        n2598 = local write "Save"(w3031) -> ()
        n2599 = local read "Main Tab"() -> (w3025:T2)
        n2600 = case shown="True" w3028 {
          frame False {
            n2601 = local read "Rt 3"() -> (w3092:bool)
            n2602 = case shown="True" w3092 {
              frame False {
              }
              frame True {
                n2603 = local write "Rt 3"(FALSE ("Rt 3")) -> ()
              }
            }
            "Rt" <- TRUE ("Rt")
            "Rt 2" <- FALSE ("Rt")
          }
          frame True {
            n2604 = local read "Rt"() -> (w3098:bool)
            n2605 = local write "Rt 2"(TRUE ("Rt 2")) -> ()
            n2606 = case shown="True" w3098 {
              frame False {
              }
              frame True {
                n2607 = local write "Rt"(FALSE ("Rt")) -> ()
              }
            }
            "Rt 3" <- TRUE ("Rt 3")
          }
        }
        n2608 = case shown="\"Acquire\"" w3025 {
          tunnel: w3027 -> [_ w3127]
          frame Default {
            w3126 = 0.0 ("output")
            n2609 = local write "PID-out"(w3126) -> ()
            n2610 = local write "Frequency ( Hz )"(w3126) -> ()
            n2611 = local write "STROKE Initialize"(TRUE ("STROKE Initialize")) -> ()
          }
          frame "Acquire" {
            n2612 = stacked-sequence {
              frame #0 {
                n2613 = local read "Auto Start Test"() -> (w3129:bool)
                n2614 = case shown="True" w3129 {
                  tunnel: "RUN" -> [w3150 w3153]
                  tunnel: [w3150 w3152] -> w3130
                  frame False {
                  }
                  frame True {
                    n2615 = local read "Auto Start Temp"() -> (w3151:bool)
                    n2616 = Or(x=w3153, y=w3151) -> (x .or. y?=w3152:bool)
                  }
                }
                n2617 = local read "clk"() -> (w3149:dbl)
                n2618 = local read "Save"() -> (w3145:bool)
                n2619 = Equal?(x=w3149, y=0.0) -> (x = y?=w3146:bool)
                n2620 = And(x=w3146, y=w3145) -> (x .and. y?=w3147:bool)
                n2621 = Not(x="Engage") -> (.not. x?=w3136:bool)
                n2622 = case shown="False" w3130 {
                  tunnel: [0.0 w3177] -> w3132
                  frame False {
                    (unwired) TRUE ("Visible")
                    n2623 = local read "Auto Start Test"() -> (w3157:bool)
                    n2624 = local write "Start Time"(TRUE ("Start Time")) -> ()
                    n2625 = property on="Stroke 2" class="DigNum (strict)"("Visible"=FALSE) -> ()  [unwired: 2 in, 2 out]
                    n2626 = case shown="False" w3157 {
                      frame False {
                        n2627 = property on="Heater Button" class="Bool (strict)"("DisabledEnum"=T19."Enabled" ("Disabled")) -> ()  [unwired: 2 in, 2 out]
                        n2628 = property on="Humidity" class="Bool (strict)"("DisabledEnum"=T19."Enabled" ("Disabled")) -> ()  [unwired: 2 in, 2 out]
                      }
                      frame True {
                      }
                    }
                    n2629 = case shown="False" "TestCompFlg" {
                      frame False {
                        n2630 = local read "StartFlg"() -> (w3165:bool)
                        n2631 = case shown="True" w3165 {
                          frame False {
                          }
                          frame True {
                            n2632 = stacked-sequence {
                              frame #0 {
                                n2633 = local read "EVENT LOG"() -> (w3169:string)
                                n2634 = call "Event Log.vi"("Content"="Test was interrupted", "EVENT LOG"=w3169) -> ("EVENT LOG"=w3170:string)  [unwired: 8 in, 1 out]
                                n2635 = local write "EVENT LOG"(w3170) -> ()
                                n2636 = property on="RUN" class="Bool (strict)"("Visible"=TRUE) -> ()  [unwired: 2 in, 2 out]
                                n2637 = property on="Auto Start Test" class="Bool (strict)"("Visible"=TRUE) -> ()  [unwired: 2 in, 2 out]
                              }
                              frame #1 {
                                w3173 = FALSE ("StartFlg")
                                n2638 = property on="Heater Button" class="Bool (strict)"("Val(Sgnl)"=FALSE ("Value (Signaling)")) -> ()  [unwired: 2 in, 2 out]
                                n2639 = local write "Heater Button"(w3173) -> ()
                                n2640 = local write "StartFlg"(w3173) -> ()
                                n2641 = local write "Humidity"(w3173) -> ()
                                n2642 = local write "Humidity 2"(TRUE ("Humidity")) -> ()
                              }
                              frame #2 {
                                n2643 = local write "Due Write"("VC;0" ("Command")) -> ()
                              }
                              frame #3 {
                                n2644 = Wait (ms)(milliseconds to wait=u32 1500) -> ()  [unwired: 1 out]
                              }
                              frame #4 {
                                n2645 = local write "Due Write"("HE;0" ("Command")) -> ()
                              }
                            }
                          }
                        }
                      }
                      frame True {
                      }
                    }
                    n2646 = local write "String 14"("Test will autostart once parameters reach the set value." ("String 14")) -> ()
                  }
                  frame True {
                    (unwired) FALSE ("Visible")
                    n2647 = property on="Stroke 2" class="DigNum (strict)"("Visible"=TRUE) -> ()  [unwired: 2 in, 2 out]
                    n2648 = property on="STOP 2" class="Bool (strict)"("Disabled"=u8 2) -> ()  [unwired: 2 in, 2 out]
                    n2649 = local write "String 14"(" Running....." ("String 14")) -> ()
                    n2650 = property on="Heater Button" class="Bool (strict)"("DisabledEnum"=T19."Disabled and Grayed Out" ("Disabled")) -> ()  [unwired: 2 in, 2 out]
                    n2651 = property on="Humidity" class="Bool (strict)"("DisabledEnum"=T19."Disabled and Grayed Out" ("Disabled")) -> ()  [unwired: 2 in, 2 out]
                    n2652 = case shown="True" "Start Time" {
                      selector: "Start Time" -> [_ w3196]
                      frame False {
                      }
                      frame True {
                        n2653 = Not(x=w3196) -> (.not. x?=w3195:bool)
                        n2654 = local write "Start Time"(w3195) -> ()
                        n2655 = local read "EVENT LOG"() -> (w3197:string)
                        n2656 = call "Event Log.vi"("Content"="Test in progress", "EVENT LOG"=w3197) -> ("EVENT LOG"=w3199:string)  [unwired: 8 in, 1 out]
                        n2657 = local write "EVENT LOG"(w3199) -> ()
                      }
                    }
                    n2658 = disable-structure shown="Enabled" {
                      disable-tunnel: [w3188 w3194] -> w3177
                      frame Disabled {
                        n2659 = local read "Set Hz"() -> (w3191:dbl)
                        n2660 = call <vilib>:"Uniform White Noise Waveform.vi"() -> ("signal out"=w3190:waveform(dbl))  [unwired: 10 in, 1 out]
                        n2661 = Random Number (0-1)() -> (number: 0 to 1=w3187:dbl)
                        n2662 = Add(x=w3191, y=w3190) -> (x+y=w3189:waveform(dbl))
                        n2663 = Multiply(x=ext 0.01 ("y"), y=w3187) -> (x*y=w3185:ext)
                        n2664 = Multiply(x=w3189, y=w3185) -> (x*y=w3188:waveform(ext))
                      }
                      frame Enabled {
                        n2665 = call-poly <vilib>:"Random Number (Range).vi"("lower bound (0)"=49.89, "upper bound (100)"=50.8) -> ("number"=w3194:dbl)  [unwired: 9 in]
                      }
                    }
                    "StartFlg" <- TRUE ("StartFlg")
                  }
                }
                n2666 = case shown="True" w3147 {
                  frame False {
                  }
                  frame True {
                    n2667 = local write "clk"(10.0 ("clk")) -> ()
                    n2668 = Get Date/Time In Seconds() -> (seconds since 1Jan1904=w3202:timestamp)
                    n2669 = To Double Precision Float(number=w3202) -> (double precision float=w3200:dbl)
                    n2670 = local write "acq timer"(w3200) -> ()
                    n2671 = local write "act save time"(w3200) -> ()
                  }
                }
                n2672 = call "Elapsed Time"("Time Target (s)"="Countdown", "Reset"=w3136) -> ("Elapsed Time (s)"=w3141:dbl, "Time has Elapsed"=w3139:bool)  [unwired: 10 in, 6 out]
                "Countdown 2" <- w3141
                n2673 = Subtract(x=w3141, y=2.0) -> (x-y=w3144:dbl)
                n2674 = Less?(x=w3144, y="Countdown") -> (x < y?=w3142:bool)
                n2675 = And(x=w3142, y=w3139) -> (x .and. y?=w3138:bool)
                n2676 = case shown="True" w3138 {
                  frame False {
                  }
                  frame True {
                    (unwired) dbl[] [] ("History Data")
                    n2677 = local write "Engage"(FALSE ("Engage")) -> ()
                    n2678 = local write "RUN"(TRUE ("RUN")) -> ()
                    n2679 = local read "Humidity ( %RH )"() -> (→"Rh Before":dbl)
                  }
                }
                n2680 = local read "Test \nStatus"() -> (w3134:bool)
                n2681 = Select(t=w3132, s=w3134, f=0.0) -> (s? t:f=w3133:dbl)
                n2682 = local write "Frequency ( Hz )"(w3133) -> ()
              }
              frame #1 {
                w3225 = 1000000.0 ("x")
                # "HC;1/0\nST;VALUE"
                # "Elapsed time\ncof\nstroke\nAir temp\nTemp\nHumidity"
                # "acq timer\n\nact save time"
                # "convert to microseconds"
                n2683 = local read "COUNT"() -> (w3208:i32)
                n2684 = local read "Rate"() -> (w3221:dbl)
                n2685 = Divide(x=w3225, y=w3221) -> (x/y=w3226:dbl)
                n2686 = Greater Or Equal?(x=w3208, y=250) -> (x >= y?=w3207:bool)
                n2687 = Get Date/Time In Seconds() -> (seconds since 1Jan1904=w3228:timestamp)
                n2688 = case shown="True" w3207 {
                  frame False {
                    n2689 = local read "COUNT"() -> (w3229:i32)
                    n2690 = Increment(x=w3229) -> (x+1=w3230:i32)
                    n2691 = local write "COUNT"(w3230) -> ()
                  }
                  frame True {
                    n2692 = local write "COUNT"(0 ("COUNT")) -> ()
                  }
                }
                n2693 = local read "Samplingtime 2"() -> (w3206:dbl)
                n2694 = local read "act save time"() -> (w3223:dbl)
                n2695 = Divide(x=w3226, y=w3225) -> (x/y=w3224:dbl)
                n2696 = To Double Precision Float(number=w3228) -> (double precision float=w3217:dbl)
                n2697 = Add(x=w3223, y=w3206) -> (x+y=w3222:dbl)
                n2698 = local read "acq timer"() -> (w3227:dbl)
                n2699 = local read "COUNT"() -> (w3210:i32)
                n2700 = Greater Or Equal?(x=w3217, y=w3222) -> (x >= y?=w3205:bool)
                n2701 = Multiply(x=w3224, y=w3210) -> (x*y=w3216:dbl)
                n2702 = Subtract(x=w3217, y=w3227) -> (x-y=w3219:dbl)
                n2703 = local read "Save"() -> (w3220:bool)
                n2704 = Add(x=w3219, y=w3216) -> (x+y=w3203:dbl)
                "Elapsed time 3" <- w3203
                n2705 = And(x=w3205, y=w3220) -> (x .and. y?=w3218:bool)
                n2706 = Divide(x=w3203, y=60.0) -> (x/y=w3214:dbl)
                n2707 = local read "Test \nStatus"() -> (w3204:bool)
                n2708 = local read "clk"() -> (w3211:dbl)
                n2709 = Equal?(x=w3211, y=10.0) -> (x = y?=w3213:bool)
                n2710 = case shown="True" w3218 {
                  tunnel: w3217 -> [_ w3344]
                  tunnel: [FALSE ("Boolean 2") TRUE ("Boolean 2")] -> _